vi "MartinsDCtest.vi"() -> ()   [LabVIEW 2011]
uses:
  Sub VIs/Trap cluster.ctl
  <vilib>/Utility/inputDevices.llb/closeKeyboard.vi
  <vilib>/Utility/inputDevices.llb/keyboardAcquire.vi
  <vilib>/Utility/file.llb/Write To Spreadsheet File (DBL).vi
  <vilib>/vision/driver/NI_Vision_Acquisition_Software.lvlib
panel:
  in  "e_desired":sgl=0.5
  in  "Apply Corrections":bool
  in  "View Licence":bool
  in  "ok":bool caption="Mark the center of \nthe spot using the \nzoom and the point\ntool, then click this \nbutton"
  in  "Stop program":bool
  in  "Updating trap cluster":bool
  out "Camera enabled":bool
  out "SLM enabled":bool
  in  "Run calibration":bool
  in  "Hologram generation":cluster{"Method":i32, "Iterations":i32}={"Method"=0, "Iterations"=10} {"Method" items=["Lenses & Gratings (3D)", " Gerchberg-Saxton (3D)", "Gerchberg-Saxton FFT (2D)"]}
  in  "Display hologram\nand computed \nimage plane":bool=TRUE
  in  "ROI":T1={"Global Rectangle"=[568, 568, 719, 569], "Contours"=[{"Contour Type"=0, "ROI Type"=1, "Points"=[568, 568]}, {"Contour Type"=0, "ROI Type"=1, "Points"=[642, 568]}, {"Contour Type"=0, "ROI Type"=1, "Points"=[718, 568]}]}
  out "Image":T2(plugin-control)
  in  "y":dbl=100.0 min=1e-22
  in  "Filename":string="test"
  out "appended path":path=path "C:/Users/Martin/Dropbox/GU/CUDA/GenerateHologramCUDA/LabVIEW/MartinDC/Measurements/test0_0.bmp"
  in  "File Path":path=path "C:/Users/Martin/Dropbox/GU/CUDA/GenerateHologramCUDA/LabVIEW/MartinDC/Measurements"
  in  "Show image":bool=TRUE
  in  "ROI size":dbl=2.0 min=2.0 step=2.0
  in  "Tab Control":enum32{"Normal", "Grid"}(tab)=enum."Grid"
  in  "Z":dbl[](array[numeric])=[0.0, 0.0, 0.0]
  in  "I":dbl[](array[numeric])=[10.0, 10.0, 10.0]
  out "#":i32[](array[numeric])=[0, 1, 2]
  in  "G":bool[](array[boolean])=[FALSE, FALSE, FALSE]
  in  "Spots y":i32=3
  in  "Grid spacing":i32=35
  in  "Spots x":i32=3
  in  "separation step":i32=1
  in  "max separation":i32=40
  in  "min separation":i32=30
  in  "Measure":bool
  in  "#images":i32=1
  out "Step number":i32
  in  "Move one spot":bool
  out "Calculated image plane":dbl[][](graph)
  out "Current trap pos":T3={"X (IMAQ)"=[555.0, 642.5, 730.0, 555.0, 642.5, 730.0, 555.0, 642.5, 730.0], "Y (IMAQ)"=[555.0, 555.0, 555.0, 642.5, 642.5, 642.5, 730.0, 730.0, 730.0], "Z"=[0.0, 0.0, 0.0, 0.0, 0.0, 0.0, 0.0, 0.0, 0.0], "Amplitudes"=[1.0, 1.0, 1.0, 1.0, 1.0, 1.0, 1.0, 1.0, 1.0], "Trap number"=[0, 1, 2, 3, 4, 5, 6, 7, 8], "ROI number"=[0, 1, 2, 3, 4, 5, 6, 7, 8], "Number of traps"=9, "Group"=[FALSE, FALSE, FALSE, FALSE, FALSE, FALSE, FALSE, FALSE, FALSE]}
  out "NI Vision error":errorcluster
  out "CUDA/SLM error":errorcluster
  in  "Cancel calibration":bool
  in  "Skip step if \ntimed out":bool
  in  "Display path":bool=TRUE
  out "Average step time (ms)":dbl
  in  "Step time \n(ms)":u32=10
  in  "Pause":bool
  in  "cancel path":bool
  out "Step skipped":bool
  in  "Path controls":T4={"follow path"=FALSE, "Step length"=1.0, "Arrive \nsimultaneously"=TRUE, "Synchronize traps"=FALSE, "Add current \npositions to path"=FALSE}
  in  "Create path":bool
  in  "Positioning  mode":enum16{"Normal", "Group", "Grid"}(ring)=enum."Grid"
  in  "Move \nHandle":bool
  out "Displayed Hologram":u8[][](graph)
  in  "Coordinate mapping \n(IMAQ to SLM)":T5={"sX"=-256.0, "sY"=-256.0, "sZ"=0.0, "cX"=0.4, "cY"=0.4, "cZ"=1.0}
  in  "Switch X/Y":bool
  # "Martin\nPersson 2011"
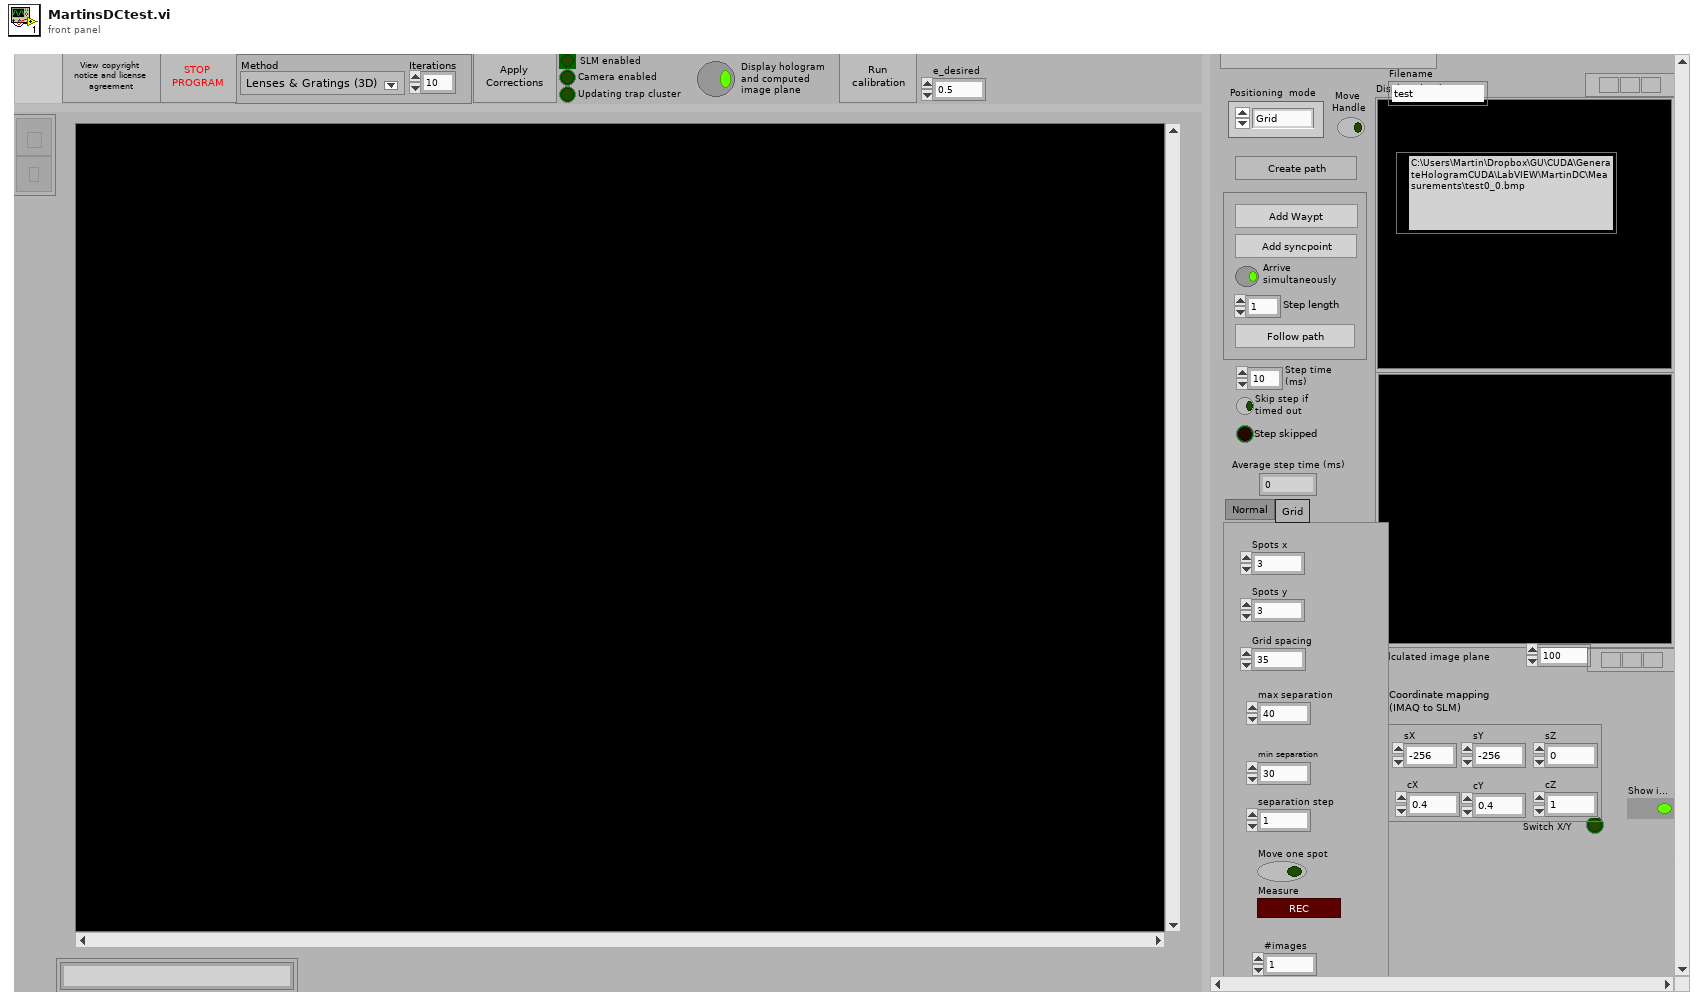
[diagram p1: front panel]
types:
  T1 = cluster{"Global Rectangle":i32[], "Contours":cluster{"Contour Type":u32, "ROI Type":u32, "Points":i32[]}[]}
  T2 = typedef "IMAQ Image.ctl" = refnum<image>
  T3 = typedef "Trap cluster.ctl" = cluster{"X (IMAQ)":dbl[], "Y (IMAQ)":dbl[], "Z":dbl[], "Amplitudes":dbl[], "Trap number":i32[], "ROI number":i32[], "Number of traps":i32, "Group":bool[]}
  T4 = cluster{"follow path":bool, "Step length":dbl, "Arrive \nsimultaneously":bool, "Synchronize traps":bool, "Add current \npositions to path":bool}
  T5 = cluster{"sX":dbl, "sY":dbl, "sZ":dbl, "cX":dbl, "cY":dbl, "cZ":dbl}
  T6 = cluster{"Centroid X":dbl[], "Centroid Y":dbl[], "Acquired Buffer Number":u32}
  T7 = typedef "IMAQdx.ctl" = refnum<k21>
  T8 = typedef "Image Type" = u32
  T9 = typedef "Semaphore RefNum" = refnum<k1>
  T10 = enum16{"0", "1", "2", "3", "4", "5", "6", "7", "8", "9", "A", "B", "C", "D", "E", "F", "G", "H", "I", "J", "K", "L", "M", "N", "O", "P", "Q", "R", "S", "T", "U", "V", "W", "X", "Y", "Z", "F1", "F2", "F3", "F4", "F5", "F6", "F7", "F8", "F9", "F10", "F11", "F12", "F13", "F14", "F15", "ADD", "BACK", "BACKSLASH", "CAPITAL", "COMMA", "DECIMAL", "DELETE", "DIVIDE", "DOWN", "END", "EQUALS", "ESCAPE", "GRAVE (`)", "HOME", "INSERT", "LBRACKET", "LCONTROL", "LEFT", "L ALT", "LSHIFT", "LWIN", "MINUS", "MULTIPLY", "NEXT", "NUMLOCK", "NUMPAD_0", "NUMPAD_1", "NUMPAD_2", "NUMPAD_3", "NUMPAD_4", "NUMPAD_5", "NUMPAD_6", "NUMPAD_7", "NUMPAD_8", "NUMPAD_9", "PAUSE", "PERIOD", "PRIOR (PG UP)", "RBRACKET", "RCONTROL", "RETURN", "RIGHT", "R ALT", "RSHIFT", "RWIN", "SCROLL", "SEMICOLON", "SLASH", "SPACE", "SUBTRACT", "TAB", "UP", "ENTER (num pad)", "' (quote)"}[]
  T11 = typedef "LVRectTypeDef.ctl" = cluster{"left":i16, "top":i16, "right":i16, "bottom":i16}
  T12 = cluster{"Contour Type":u32, "ROI Type":u32, "Points":i32[]}[]
  T13 = cluster{"Contour Type":u32, "ROI Type":u32, "Points":i32[]}
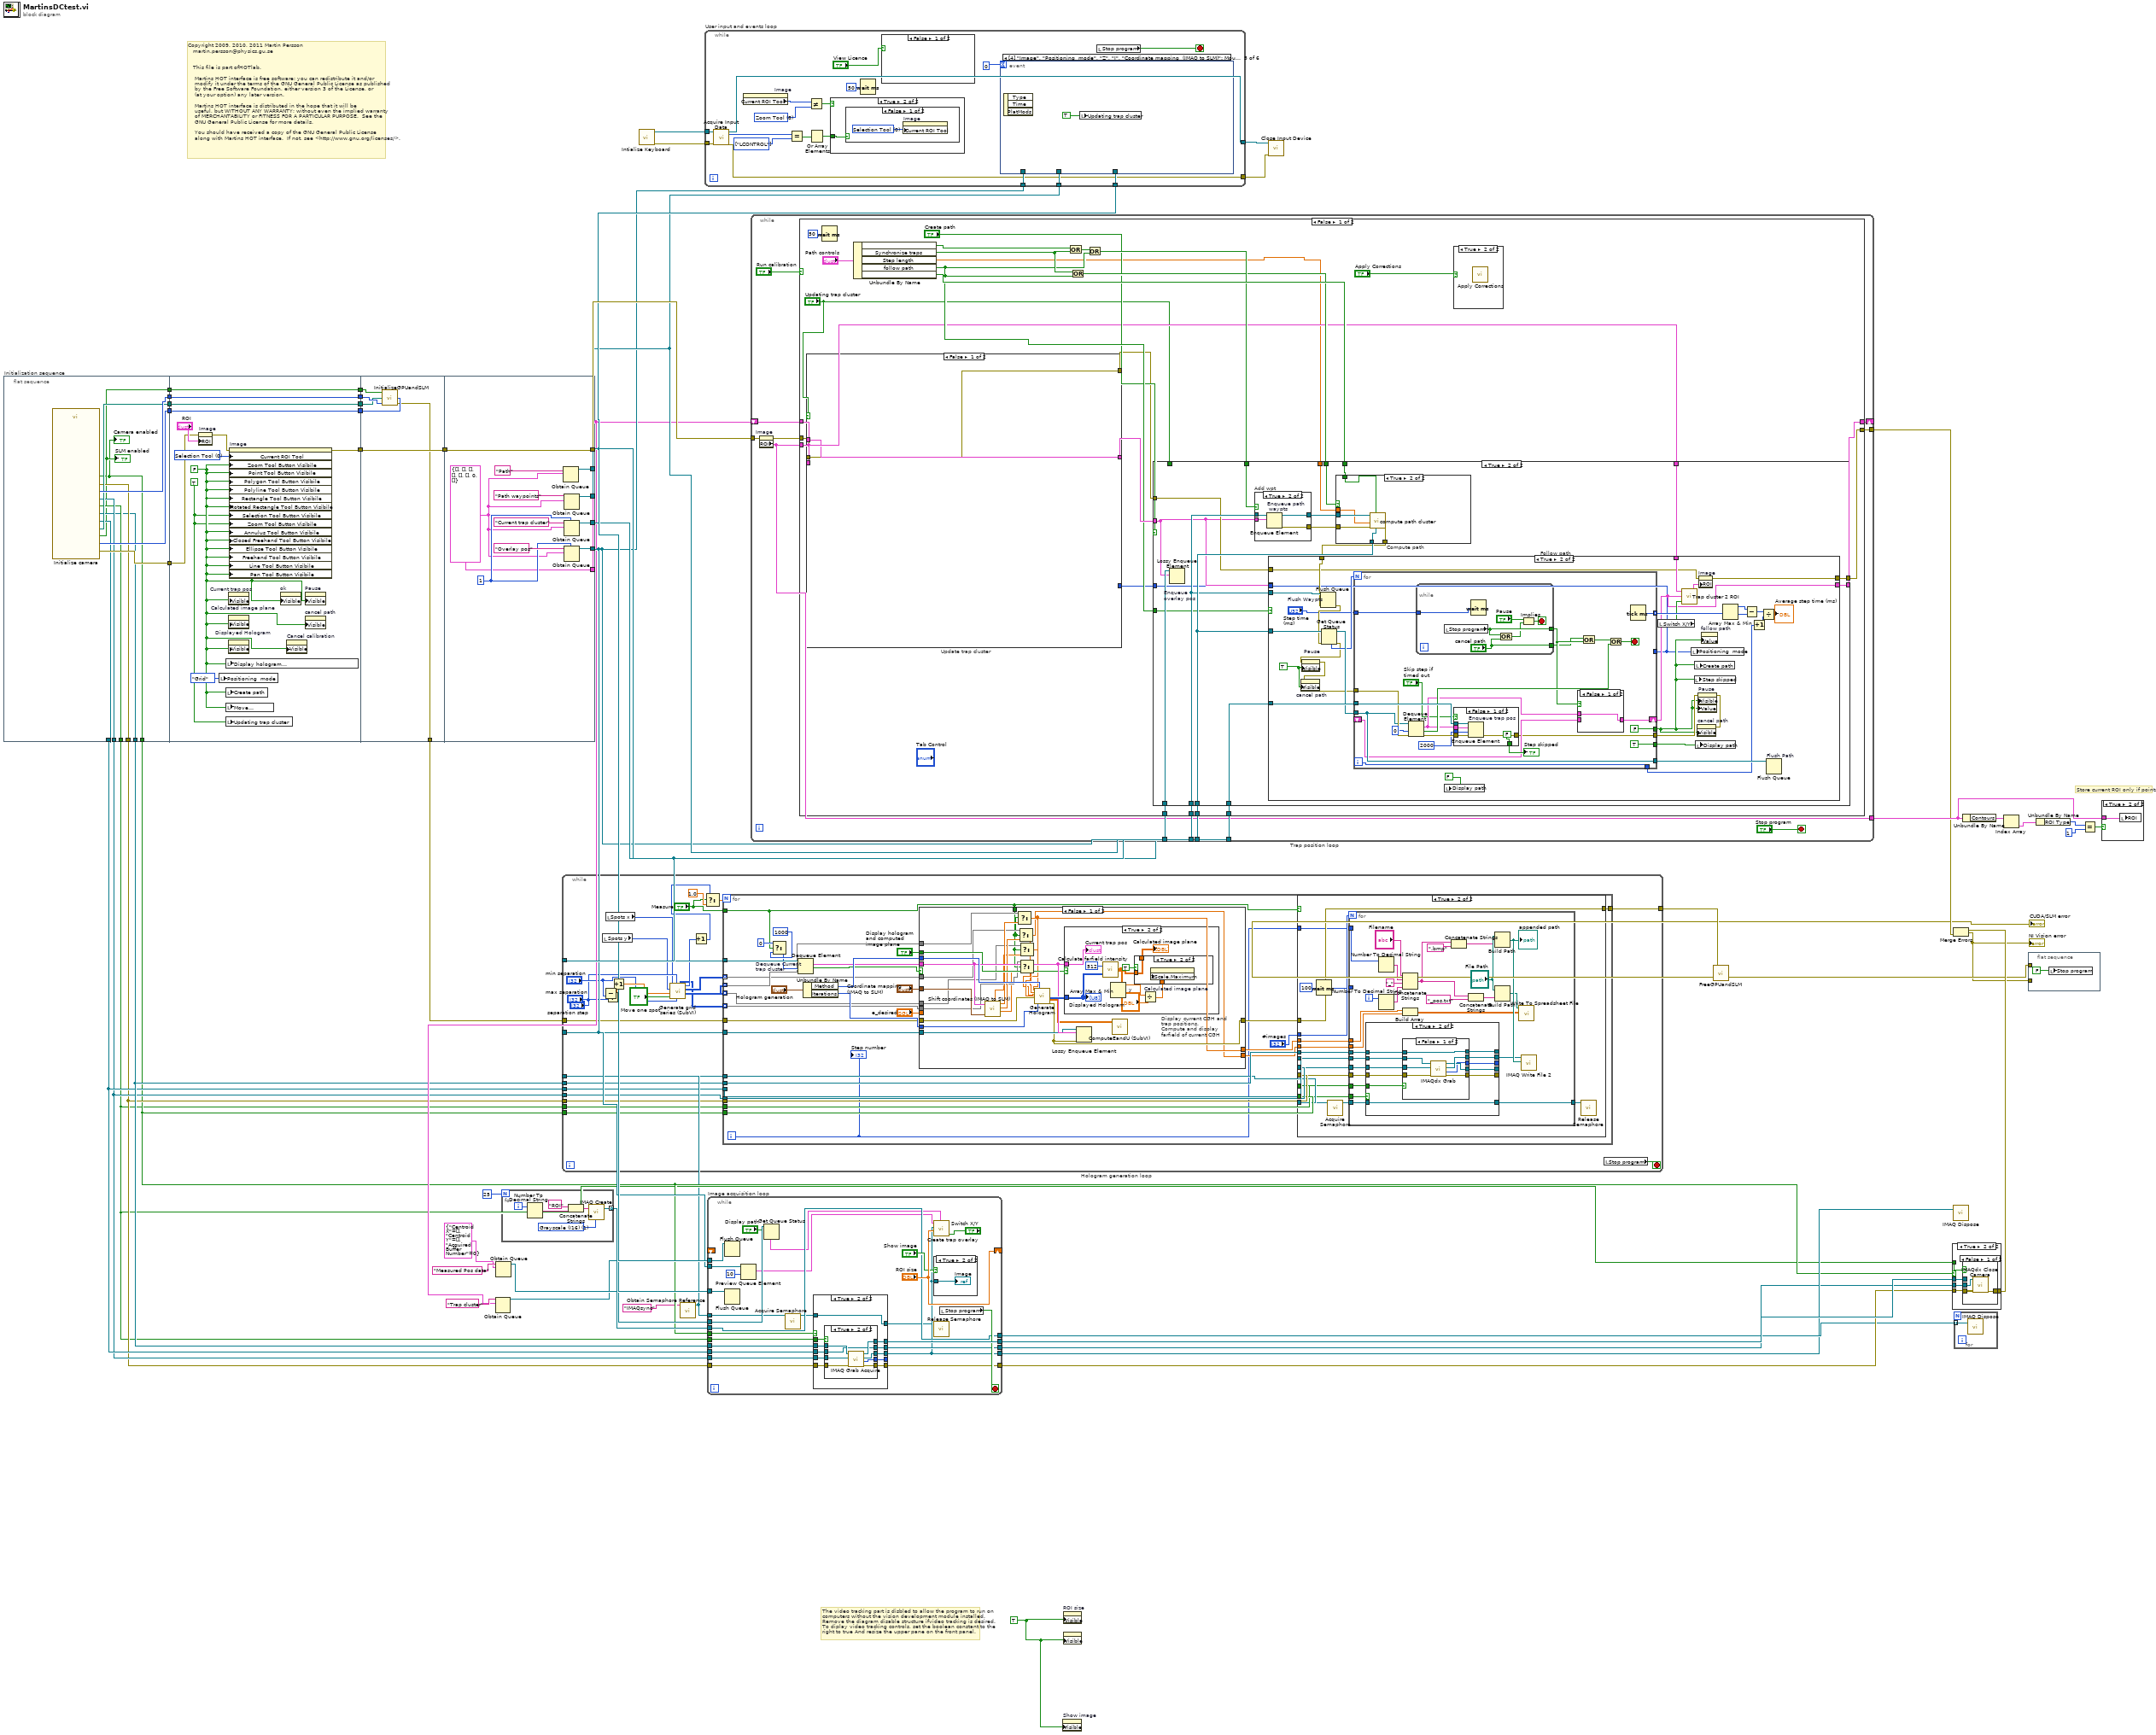
[diagram p0: block diagram]
diagram:
  w41 = TRUE ("Visible")
  # "Copyright 2009, 2010, 2011 Martin Persson \n   martin.persson@physics.gu.se\n\n\n   This file is part ofHOTlab.\n\n    Martins HOT interface is free software: you can redistribute it and/or \n    modify it under the terms of the GNU General Public License as published \n    by the Free Software Foundation, either version 3 of the License, or\n    (at your option) any later version.\n\n    Martins HOT interface is distributed in the hope that it will be \n    useful, but WITHOUT ANY WARRANTY; without even the implied warranty\n    of MERCHANTABILITY or FITNESS FOR A PARTICULAR PURPOSE.  See the\n    GNU General Public License for more details.\n\n    You should have received a copy of the GNU General Public License\n    along with Martins HOT interface.  If not, see <http://www.gnu.org/licenses/>."
  # "Store current ROI only if points"
  # "The video tracking part is disbled to allow the program to run on\ncomputers without the vision development module installed. \nRemove the diagram disable structure ifvideo tracking is desired. \nTo diplay video tracking controls, set the boolean constant to the \nright to true And resize the upper pane on the front panel."
  n1 = flat-sequence "Initialization sequence" {
    tunnel: [w56] -> w26
    tunnel: [w65] -> w25
    tunnel: [w64] -> w24
    tunnel: [w63] -> w23
    tunnel: [w62] -> w22
    tunnel: [w61] -> w6
    tunnel: [w60] -> w7
    tunnel: [w59] -> w5
    tunnel: [w58] -> w3
    tunnel: [w57] -> w8
    tunnel: [w55] -> w4
    tunnel: w26 -> [w74]
    tunnel: w25 -> [w72]
    tunnel: w24 -> [w77]
    tunnel: w23 -> [w76]
    tunnel: w22 -> [w75]
    tunnel: [w74] -> w15
    tunnel: [w67] -> w14
    tunnel: [w77] -> w12
    tunnel: [w76] -> w11
    tunnel: [w75] -> w10
    tunnel: w15 -> [w80]
    tunnel: w14 -> [w83]
    tunnel: [w83] -> w13
    tunnel: w12 -> [w81]
    tunnel: w11 -> [w82]
    tunnel: w10 -> [w79]
    tunnel: [w78] -> w9
    tunnel: [w94] -> w21
    tunnel: w13 -> [w94]
    tunnel: [w92] -> w20
    tunnel: [w90] -> w19
    tunnel: [w88] -> w18
    tunnel: [w87] -> w17
    tunnel: [w84] -> w16
    frame #0 {
      n2 = call "Initialize camera.vi"() -> ("CUDA device ID"=w63:i32, "IMAQdx Session Out"=w60:T7, "TrueFrame out"=w64:i32, "IMAQ camera"=w58:bool, "Image reference out"=w61:T2, "SLM enabled"=w56:bool, "Camera enabled"=w55:bool, "Vision error out"=w65:errorcluster, "LUT path out"=w62:path, "IMAQ Session Out"=w57:refnum<k11>, "Camera error"=w59:errorcluster)  [unwired: 5 in]
      "Camera enabled" <- w55
      "SLM enabled" <- w56
    }
    frame #1 {
      w70 = TRUE ("ROI Tool Buttons Visibile:Zoom Tool Button Visible")
      w71 = FALSE ("ROI Tool Buttons Visibile:Zoom Tool Button Visible")
      w69 = u32 0 items=["Zoom Tool"=8, "Selection Tool"=0, "Pan Tool"=9, "Point Tool"=1, "Line Tool"=2, "Rectangle Tool"=3, "Rotated Rectangle Tool"=12, "Polyline Tool"=10, "Polygon Tool"=5, "Freehand Tool"=11, "Closed Freehand Tool"=6, "Ellipse Tool"=4, "Annulus Tool"=7] ("Current ROI Tool")
      n3 = property on="Image" class="ImageControl"(error in=w72, "ROI"="ROI") -> (error out=w68:errorcluster)  [unwired: 1 in, 1 out]
      n4 = local write "Positioning  mode"(enum16{"Normal", "Group", "Grid"}."Grid" ("Positioning  mode")) -> ()
      n5 = local write "Display hologram\nand computed \nimage plane"(w71) -> ()
      n6 = local write "Create path"(w71) -> ()
      n7 = local write "Move \nHandle"(w71) -> ()
      n8 = local write "Updating trap cluster"(w70) -> ()
      n9 = property on="Current trap pos" class="Clust (strict)"("Visible"=w71) -> ()  [unwired: 2 in, 2 out]
      n10 = property on="Calculated image plane" class="IntGraph (strict)"("Visible"=w71) -> ()  [unwired: 2 in, 2 out]
      n11 = property on="Displayed Hologram" class="IntGraph (strict)"("Visible"=w71) -> ()  [unwired: 2 in, 2 out]
      n12 = property on="Image" class="ImageControl"(error in=w68, "Current ROI Tool"=w69, "Zoom Tool Button Visibile"=w71, "Point Tool Button Visibile"=w71, "Polygon Tool Button Visibile"=w71, "Polyline Tool Button Visibile"=w71, "Rectangle Tool Button Visibile"=w71, "Rotated Rectangle Tool Button Visibile"=w71, "Selection Tool Button Visibile"=w70, "Zoom Tool Button Visibile"=w70, "Annulus Tool Button Visibile"=w71, "Closed Freehand Tool Button Visibile"=w71, "Ellipse Tool Button Visibile"=w71, "Freehand Tool Button Visibile"=w71, "Line Tool Button Visibile"=w71, "Pan Tool Button Visibile"=w71) -> (error out=w67:errorcluster)  [unwired: 1 in, 1 out]
      n13 = property on="ok" class="Bool"("Visible"=w71) -> ()  [unwired: 2 in, 2 out]
      n14 = property on="Cancel calibration" class="Bool"("Visible"=w71) -> ()  [unwired: 2 in, 2 out]
      n15 = property on="Pause" class="Bool (strict)"("Visible"=w71) -> ()  [unwired: 2 in, 2 out]
      n16 = property on="cancel path" class="Bool"("Visible"=w71) -> ()  [unwired: 2 in, 2 out]
    }
    frame #2 {
      n17 = call "InitializeGPUandSLM.vi"("TrueFrame"=w81, "deviceId"=w82, "Path to LUT file"=w79, "SLM enabled"=w80) -> ("CUDA/SLM error"=w78:errorcluster)  [unwired: 1 out]
    }
    frame #3 {
      w85 = 1 ("max queue size (-1, unlimited)")
      w84 = T3 {"X (IMAQ)"=[], "Y (IMAQ)"=[], "Z"=[], "Amplitudes"=[], "Trap number"=[], "ROI number"=[], "Number of traps"=0, "Group"=[]} ("output cluster 2")
      n18 = Obtain Queue(name (unnamed)="Path", element data type=w84) -> (queue out=w92:refnum<queue>)  [unwired: 3 in, 2 out]
      n19 = Obtain Queue(name (unnamed)="Path waypoints", element data type=w84) -> (queue out=w90:refnum<queue>)  [unwired: 3 in, 2 out]
      n20 = Obtain Queue(max queue size (-1, unlimited)=w85, name (unnamed)="Current trap cluster", element data type=w84) -> (queue out=w88:refnum<queue>)  [unwired: 2 in, 2 out]
      n21 = Obtain Queue(max queue size (-1, unlimited)=w85, name (unnamed)="Overlay pos", element data type=w84) -> (queue out=w87:refnum<queue>)  [unwired: 2 in, 2 out]
    }
  }
  n22 = Obtain Queue(name (unnamed)="Trap cluster", element data type=w16) -> (queue out=w46:refnum<queue>)  [unwired: 3 in, 2 out]
  n23 = Obtain Queue(name (unnamed)="Measured Pos data", element data type=T6 {"Centroid X"=[], "Centroid Y"=[], "Acquired Buffer Number"=0} ("output cluster 2")) -> (queue out=w49:refnum<queue>)  [unwired: 3 in, 2 out]
  n24 = for {
    N: 25 -> [_]
    tunnel: [w100] -> w51 mode=indexing
    i -> [w96]
    w98 = T8 1 items=["Grayscale (U8)", "Grayscale (I16)", "Grayscale (SGL)", "Complex (CSG)", "RGB (U32)", "HSL (U32)", "RGB (U64)", "Grayscale (U16)"] ("Image Type")
    n25 = Number To Decimal String(number=w96) -> (decimal integer string=w95:string)  [unwired: 1 in]
    n26 = Concatenate Strings("ROI" ("Image Name"), w95) -> (w97:string)
    n27 = call "IMAQ Create"("Image Name"=w97, "Image Type"=w98) -> ("New Image"=w100:T2)  [unwired: 3 in, 1 out]
  }
  n28 = call <vilib>:"Intialize Keyboard.vi"() -> ("error out"=w28:errorcluster, "device ID"=w54:refnum<k1>)  [unwired: 1 in, 9 out]
  n29 = call <vilib>:"Obtain Semaphore Reference.vi"("name (unnamed)"="IMAQsync") -> ("semaphore"=w1:T9)  [unwired: 4 in, 2 out]
  n30 = while "Hologram generation loop" {
    tunnel: w18 -> [w129]
    tunnel: w17 -> [w127]
    tunnel: w9 -> [w128]
    tunnel: [w122] -> w32
    tunnel: w8 -> [w126]
    tunnel: w7 -> [w125]
    tunnel: w6 -> [w124]
    tunnel: w5 -> [w123]
    tunnel: w4 -> [w121]
    tunnel: w3 -> [w120]
    tunnel: w1 -> [w119]
    stop <- w130 stop-if-true
    n31 = local read "Spots y"() -> (w108:i32)
    n32 = Subtract(x="max separation", y="min separation") -> (x-y=w114:i32)
    n33 = Divide(x=w114, y="separation step") -> (x/y=w113:dbl)
    n34 = local read "Spots x"() -> (w109:i32)
    n35 = Increment(x=w113) -> (x+1=w112:dbl)
    n36 = call "Generate grid series (SubVI).vi"("min separation"="min separation", "separation step"="separation step", "Move one spot"="Move one spot", "Number of steps"=w112, "Spots y"=w108, "Spots x"=w109) -> ("Y"=w105:i32[][], "X"=w104:i32[][], "Numeric out"=w107:i32, "Z"=w103:i32[][], "I"=w102:i32[][])  [unwired: 1 in]
    n37 = Increment(x=w107) -> (x+1=w106:i32)
    n38 = Select(t=w106, s="Measure", f=1.0) -> (s? t:f=w118:dbl)
    n39 = for {
      N: w118 -> [_]
      tunnel: w129 -> [w160]
      tunnel: w128 -> [w155]
      tunnel: w127 -> [w153]
      tunnel: w126 -> [w151]
      tunnel: w125 -> [w150]
      tunnel: w124 -> [w149]
      tunnel: w123 -> [w148]
      tunnel: [w146] -> w122
      tunnel: w121 -> [w143]
      tunnel: w120 -> [w142]
      tunnel: w119 -> [w140]
      tunnel: "Measure" -> [w132]
      tunnel: w105 -> [w136] mode=indexing
      tunnel: w104 -> [w135] mode=indexing
      tunnel: w103 -> [w134] mode=indexing
      tunnel: w102 -> [w133] mode=indexing
      i -> [w131]
      n40 = Select(t=0, s=w132, f=1000 ("timeout in ms (-1)")) -> (s? t:f=w137:i32)
      n41 = Dequeue Element "Dequeue Current \ntrap cluster"(queue=w160, timeout in ms (-1)=w137) -> (element=w159:T3, timed out?=w141:bool)  [unwired: 1 in, 2 out]
      n42 = Unbundle By Name("Hologram generation") -> ("Method"=w162:i32, "Iterations"=w161:i32)
      n43 = case shown="False" w141 {
        tunnel: "Coordinate mapping \n(IMAQ to SLM)" -> [w261 _]
        tunnel: "Display hologram\nand computed \nimage plane" -> [w255 _]
        tunnel: w162 -> [w259 _]
        tunnel: w161 -> [w258 _]
        tunnel: w159 -> [w257 _]
        tunnel: w153 -> [w256 _]
        tunnel: w155 -> [w254 w273]
        tunnel: [w253 w273] -> w147
        tunnel: "e_desired" -> [_ _]
        tunnel: [w241 _] -> w145
        tunnel: [w240 _] -> w144
        tunnel: w136 -> [w250 _]
        tunnel: w135 -> [w249 _]
        tunnel: w134 -> [w248 _]
        tunnel: w133 -> [w247 _]
        tunnel: w132 -> [w242 _]
        frame False {
          n44 = call "Shift coordinates (IMAQ to SLM).vi"("Trap cluster"=w257, "Coordinate mapping \n(IMAQ to SLM)"=w261) -> ("X (SLM)"=w252:sgl[], "Y (SLM)"=w251:sgl[], "Intensities"=w245:sgl[], "Z (SLM)"=w244:sgl[])  [unwired: 1 in, 1 out]
          n45 = Select(t=w250, s=w242, f=w252) -> (s? t:f=w241:sgl[])
          n46 = Select(t=w249, s=w242, f=w251) -> (s? t:f=w240:sgl[])
          n47 = Select(t=w248, s=w242, f=w244) -> (s? t:f=w243:sgl[])
          n48 = Select(t=w247, s=w242, f=w245) -> (s? t:f=w246:sgl[])
          n49 = call "Generate Hologram.vi"("x"=w241, "y"=w240, "z"=w243, "spot_intensities"=w246, "CUDA/SLM error in"=w254, "N_iterations"=w258, "method"=w259) -> ("CGH out"=w260:u8[][], "weights"=w239:sgl[][], "CUDA/SLM error out"=w253:errorcluster)  [unwired: 17 in, 1 out]
          n50 = case "Display current CGH and trap positions.\nCompute and display farfield of current CGH" shown="True" w255 {
            tunnel: w260 -> [_ w270]
            tunnel: w257 -> [_ w269]
            frame False {
            }
            frame True {
              n51 = call "Calculate farfield intensity.vi"("h_pSLM"=w270, "Numeric"=512) -> ("Calculated image plane"=w264:dbl[][])
              n52 = Array Max & Min(array=w264) -> (max value=w267:dbl)  [unwired: 3 out]
              n53 = Divide(x=w267, y="y") -> (x/y=w265:dbl)
              n54 = case shown="True" TRUE {
                tunnel: w265 -> [_ w272]
                tunnel: w264 -> [_ w271]
                tunnel: [_ w271] -> w263
                frame False {
                }
                frame True {
                  n55 = property on="Calculated image plane" class="IntGraph (strict)"("ZScale.Maximum"=w272) -> ()  [unwired: 2 in, 2 out]
                }
              }
              "Calculated image plane" <- w263
              "Displayed Hologram" <- w270
              "Current trap pos" <- w269
            }
          }
          n56 = Lossy Enqueue Element(queue=w256, element=w257, error in (no error)=w253) -> ()  [unwired: 4 out]
          n57 = call "ComputeEandU (SubVI).vi"("weights in"=w239) -> ()  [unwired: 9 in, 2 out]
        }
        frame True {
        }
      }
      n58 = case shown="True" w132 {
        tunnel: "#images" -> [_ w179]
        tunnel: w151 -> [_ w178]
        tunnel: w150 -> [_ w177]
        tunnel: w149 -> [_ w176]
        tunnel: w148 -> [_ w175]
        tunnel: w140 -> [_ w174]
        tunnel: w147 -> [w163 w171]
        tunnel: [w163 w171] -> w146
        tunnel: w145 -> [_ w170]
        tunnel: w144 -> [_ w169]
        tunnel: w143 -> [_ w168]
        tunnel: w142 -> [_ w167]
        tunnel: w131 -> [_ w166]
        frame False {
        }
        frame True {
          n59 = Wait (ms)(milliseconds to wait=u32 100) -> (millisecond timer value=w165:u32)
          n60 = call <vilib>:"Acquire Semaphore.vi"("semaphore"=w174) -> ("semaphore out"=w173:T9)  [unwired: 4 in, 2 out]
          n61 = for {
            N: w179 -> [_]
            tunnel: w178 -> [w193]
            tunnel: w177 -> [w192]
            tunnel: w176 -> [w191]
            tunnel: w175 -> [w190]
            tunnel: w173 -> [w189]
            tunnel: [w188] -> w172
            tunnel: w170 -> [w186]
            tunnel: w169 -> [w185]
            tunnel: w168 -> [w183]
            tunnel: w167 -> [w182]
            tunnel: w166 -> [w180]
            tunnel: w165 -> [_]
            i -> [w184]
            n62 = case shown="True" w183 {
              tunnel: w191 -> [w210 w222]
              tunnel: w193 -> [w209 w221]
              tunnel: [w209 w220] -> _
              tunnel: [w208 w219] -> _
              tunnel: [w210 w218] -> w187
              tunnel: [w211 w217] -> _
              tunnel: w192 -> [w211 w216]
              tunnel: w182 -> [_ w215]
              tunnel: w190 -> [w208 w214]
              tunnel: [_ w213] -> _
              tunnel: w189 -> [w206 w212]
              tunnel: [w206 w212] -> w188
              frame False {
                n63 = Wait (ms)(milliseconds to wait=u32 100) -> ()  [unwired: 1 out]
              }
              frame True {
                n64 = case shown="False" w215 {
                  tunnel: w222 -> [w230 w238]
                  tunnel: [w228 w237] -> w220
                  tunnel: [w227 w236] -> w219
                  tunnel: w221 -> [w228 w235]
                  tunnel: [w229 w234] -> w218
                  tunnel: [w224 w233] -> w213
                  tunnel: [w226 w232] -> w217
                  tunnel: w216 -> [w225 w232]
                  tunnel: w214 -> [w223 w231]
                  frame False {
                    n65 = call <vilib>:"IMAQdx Grab.vi"("error in"=w223, "Image In"=w230, "Session In"=w225) -> ("error out"=w227:errorcluster, "Buffer Number Out"=w224:u32, "Image Out"=w229:T2, "Session Out"=w226:T7)  [unwired: 5 in]
                  }
                  frame True {
                    n66 = call <vilib>:"IMAQ Grab Acquire.vi"("error in (no error)"=w231, "Image In"=w238, "IMAQ Session In"=w235) -> ("error out"=w236:errorcluster, "Acquired Buffer Number"=w233:u32, "Image Out"=w234:T2, "IMAQ Session Out"=w237:refnum<k11>)  [unwired: 1 in, 4 out]
                  }
                }
              }
            }
            n67 = Number To Decimal String(number=w180) -> (decimal integer string=w196:string)  [unwired: 1 in]
            n68 = Number To Decimal String(number=w184) -> (decimal integer string=w198:string)  [unwired: 1 in]
            n69 = Concatenate Strings("Filename", w196, "_" ("string"), w198) -> (w200:string)
            n70 = Build Array(w186, w185) -> (w181:sgl[][])
            n71 = Concatenate Strings(w200, ".bmp" ("string")) -> (w202:string)
            n72 = Concatenate Strings(w200, "_pos.txt" ("string")) -> (w205:string)
            n73 = Build Path(base path="File Path", name or relative path=w202) -> (appended path=w195:path)
            "appended path" <- w195
            n74 = Build Path(base path="File Path", name or relative path=w205) -> (appended path=w194:path)
            n75 = call-poly <vilib>:"Write To Spreadsheet File.vi"("2D data"=w181, "file path (dialog if empty)"=w194) -> ()  [unwired: 6 in, 1 out]
            n76 = call-poly "IMAQ Write File 2"("File Path"=w195, "Image"=w187) -> ()  [unwired: 8 in, 2 out]
          }
          n77 = call <vilib>:"Release Semaphore.vi"("semaphore"=w172) -> ()  [unwired: 5 in, 2 out]